vi "run_pharmaBotExp_v0.015.vi"(0 "data in":T12={"daq_ao 1"="Dev1/ao0", "daq_ai 1"="Dev1/ai0", "experiment day folder"=path "C:/multiBot/data/debug/testing", "Multiclamp init error"=0, "Multiclamp Handle Out"=10225184, "sampling rate (Hz)"=20000, "trial name"="t1"}, 1 "auto run?":bool=TRUE, 3 "which manipulator":T13(ring), 4 "HEK/slice options":enum16{"slice", "HEK"}(ring), 5 "error in":errorcluster, 6 "Validate after Experiment":bool, 7 "common cluster":T9, 11 "individual controls in":T8, 13 "images":T3={"slice image"="remote image 000000001461186C", "pipette template"="remote image 000000001461152C", "found pipette"=refnum, "pipette mask for cell tracker"=refnum, "cell images ref"=refnum}) -> (10 "Cell Looks Good?":bool=TRUE, 12 "ValidationOutputCluster":T5(array[cluster]), 14 "ValidationResults":waveform(dbl)[][](array[waveform]), 15 "ValidationPos1":T6(array[ring]), 16 "Exp. Terminated":bool, 17 "ValidationPos2":T6(array[ring]), 18 "ValidationWaveform":waveform(dbl)[](array[waveform]), 19 "error out":errorcluster)   [LabVIEW 2015] (continued)
          }
        }
        n1077 = Select(t="QualityCheck" ("ExpPhase"), s=w837, f="postLift" ("ExpPhase")) -> (s? t:f=w864:string)
        n1078 = call "run_repeatingMembraneTest_pharmabot.vi"("ExpPhase"=w864, "error in"=w900, "data in"=w899, "misc common.stop memtest"=w885, "controls array in"=w893) -> ("error out"=w897:errorcluster, "data out"=w898:T12, "Cell Good?"=w859:bool, "control array out"=w892:refnum<vi>[])  [unwired: 2 in, 1 out]
        n1079 = local write "Cell Looks Good?"(w859) -> ()
        n1080 = case shown="True" w859 {
          tunnel: w898 -> [w1208 w1260]
          tunnel: w897 -> [w1206 w1257]
          tunnel: w824 -> [_ w1235]
          tunnel: w833 -> [_ w1251]
          tunnel: w895 -> [_ w1250]
          tunnel: w894 -> [_ w1249]
          tunnel: w892 -> [w1203 w1248]
          tunnel: [w1208 w1244] -> w891
          tunnel: [w1205 w1225] -> w890
          tunnel: [w1204 w1226] -> w889
          tunnel: w885 -> [_ w1222]
          tunnel: w880 -> [_ w1241]
          tunnel: w879 -> [_ w1240]
          tunnel: w883 -> [w1201 _]
          tunnel: [w1195 w1231] -> w876
          tunnel: [w1198 w1233] -> w875
          tunnel: [w1194 w1232] -> w874
          tunnel: [w1196 w1230] -> w873
          tunnel: [w1197 w1229] -> w872
          tunnel: w837 -> [_ w1224]
          tunnel: w858 -> [_ w1218]
          frame False {
            n1081 = local read "ValidationOutputCluster"() -> (w1197:T5)
            n1082 = local read "ValidationWaveform"() -> (w1196:waveform(dbl)[])
            n1083 = local read "ValidationPos2"() -> (w1194:T6)
            n1084 = local read "ValidationPos1"() -> (w1198:T6)
            n1085 = local read "ValidationResults"() -> (w1195:waveform(dbl)[][])
            n1086 = call <vilib>:"Play Sound File.vi"("path"=path "C:/multiBot/patcherBot/sounds/Price_Is_Right_loser_clip.wav") -> ()  [unwired: 9 in, 2 out]
            n1087 = Select(t="Cell Lift Failed!" ("status string in"), s=w1201, f="Pulling Patch Failed!" ("status string in")) -> (s? t:f=w1202:string)
            n1088 = call "set_status_string.vi"("error in"=w1206, "new line?"=TRUE, "status string in"=w1202, "controls array"=w1203) -> ("error out"=w1205:errorcluster, "controls array out"=w1204:refnum<vi>[])  [unwired: 6 in]
          }
          frame True {
            n1089 = local read "How Many Experimental Phases?"() -> (w1234:i32)
            n1090 = local write "protocol creation"(T11."Experimental Procedures" ("protocol creation")) -> ()
            n1091 = case shown="True" w1224 {
              tunnel: w1257 -> [w1324 w1327]
              tunnel: [w1323 w1326] -> w1256
              tunnel: T42."Experiment Safe Position" ("Which Jumper Position to Set?") -> [w1322 _]
              tunnel: w1251 -> [w1321 _]
              tunnel: w1249 -> [w1320 _]
              tunnel: w1248 -> [w1319 w1329]
              tunnel: [w1318 w1328] -> w1247
              frame False {
                n1092 = call "moveToJumperPosition-v02.vi"("which manipulator"=w1320, "controls array in"=w1319, "Which Jumper Position to move to?"=w1322, "error in"=w1324, "common cluster"=w1321) -> ("control array out"=w1318:refnum<vi>[], "error out"=w1323:errorcluster)  [unwired: 9 in]
              }
              frame True {
                n1093 = call "set_status_string.vi"("error in"=w1327, "new line?"=TRUE, "status string in"="Not Moving", "controls array"=w1329) -> ("error out"=w1326:errorcluster, "controls array out"=w1328:refnum<vi>[])  [unwired: 6 in]
              }
            }
            n1094 = call "run_repeatingMembraneTest_pharmabot.vi"("ExpPhase"="preQC", "error in"=w1256, "data in"=w1260, "misc common.stop memtest"=w1222, "controls array in"=w1247) -> ("error out"=w1239:errorcluster, "data out"=w1258:T12, "Cell Good?"=w1221:bool, "control array out"=w1259:refnum<vi>[])  [unwired: 2 in, 1 out]
            n1095 = call "mclamp_zero_pipetteCap.vi"("error in (no error)"=w1239, "Error in"=w1240, "Multiclamp Handle Out"=w1241) -> ("error out"=w1238:errorcluster, "slow comp (pF)"=w1236:dbl, "fast comp (pF)"=w1237:dbl)  [unwired: 6 in]
            n1096 = local write "Cell Looks Good?"(w1221) -> ()
            n1097 = local write "slow comp (pF)"(w1236) -> ()
            n1098 = local write "fast comp (pF)"(w1237) -> ()
            n1099 = call "run_repeatingMembraneTest_pharmabot.vi"("ExpPhase"="preExp", "error in"=w1238, "data in"=w1258, "misc common.stop memtest"=w1222, "controls array in"=w1259) -> ("error out"=w1253:errorcluster, "data out"=w1245:T12, "Cell Good?"=w1220:bool, "control array out"=w1254:refnum<vi>[])  [unwired: 2 in, 1 out]
            n1100 = for {
              N: w1234 -> [_]
              tunnel: w1251 -> [w1334]
              tunnel: w1250 -> [w1335]
              tunnel: [w1345] -> w1246
              tunnel: w1254 -> [w1353]
              tunnel: w1249 -> [w1352]
              tunnel: w1235 -> [w1349]
              tunnel: w1253 -> [w1339]
              tunnel: [w1344] -> w1252
              tunnel: w1245 -> [w1350]
              tunnel: w1224 -> [w1348]
              shift-right: [w1346] -> _
              shift-left: FALSE ("Cell Good?") -> [w1347]
              tunnel: w1222 -> [w1343]
              tunnel: w1218 -> [w1342]
              tunnel: [w1332] -> w1217
              i -> [w1351]
              n1101 = Unbundle By Name(w1334) -> ("misc common.Terminate Experiment"=w1333:refnum<vi>)
              n1102 = control-ref of="Terminate Experiment"() -> (w1336:refnum<vi>)
              n1103 = control-ref of="Filtered currents (pA)"() -> (w1340:refnum<vi>)
              n1104 = property class="Bool (strict)"(reference=w1333) -> ("Value"=w1332:bool)  [unwired: 1 in, 2 out]
              n1105 = property class="WFGraph (strict)"(reference=w1340, error in=w1339, "Value"=waveform(dbl)[] []) -> (error out=w1338:errorcluster)  [unwired: 1 out]
              n1106 = property class="Bool (strict)"(reference=w1336, "Value"=w1332) -> ()  [unwired: 1 in, 2 out]
              n1107 = local read "current clamp"() -> (w1331:enum16{"VClamp", "IClamp"})
              n1108 = Or(x=w1332, y=w1347) -> (x .or. y?=w1341:bool)
              n1109 = case shown="False" w1341 {
                selector: w1341 -> [_ w1578]
                tunnel: w1334 -> [w1394 _]
                tunnel: w1335 -> [w1393 _]
                tunnel: w1353 -> [w1392 w1584]
                tunnel: w1352 -> [w1391 _]
                tunnel: w1338 -> [w1390 w1582]
                tunnel: w1351 -> [w1388 w1579]
                tunnel: w1350 -> [w1377 _]
                tunnel: w1349 -> [w1370 _]
                tunnel: w1348 -> [w1384 _]
                tunnel: [w1382 w1578] -> w1346
                tunnel: [w1379 w1577] -> w1345
                tunnel: [w1367 w1576] -> w1344
                tunnel: w1343 -> [w1376 _]
                tunnel: w1342 -> [w1371 _]
                tunnel: w1331 -> [w1358 _]
                frame False {
                  n1110 = Increment(x=w1388) -> (x+1=w1369:i32)
                  n1111 = case shown="1" w1369 {
                    tunnel: w1370 -> [w1502 w1508 w1514 w1520 w1526 w1532 w1538 w1544 w1550 w1556 w1562 w1568 w1574]
                    tunnel: [w1501 w1507 w1513 w1519 w1525 w1531 w1537 w1543 w1549 w1555 w1561 w1567 w1573] -> w1364
                    tunnel: w1390 -> [w1500 w1505 w1511 w1517 w1523 w1529 w1535 w1541 w1547 w1553 w1559 w1565 w1571]
                    tunnel: [w1500 w1505 w1511 w1517 w1523 w1529 w1535 w1541 w1547 w1553 w1559 w1565 w1571] -> w1389
                    tunnel: ["na" "A" "B" "C" "D" "E" "F" "G" "H" "I" "J" "K" "L"] -> w1355
                    tunnel: [w1498 w1504 w1510 w1516 w1522 w1528 w1534 w1540 w1546 w1552 w1558 w1564 w1570] -> w1361
                    tunnel: [T19."PhaseA" ("Experimental Phases") T19."PhaseA" ("Experimental Phases") T19."PhaseB" ("Experimental Phases") T19."PhaseC" ("Experimental Phases") T19."PhaseD" ("Experimental Phases") T19."PhaseE" ("Experimental Phases") T19."PhaseF" ("Experimental Phases") T19."PhaseG" ("Experimental Phases") T19."PhaseH" ("Experimental Phases") T19."PhaseI" ("Experimental Phases") T19."PhaseJ" ("Experimental Phases") T19."PhaseK" ("Experimental Phases") T19."PhaseL" ("Experimental Phases")] -> w1359
                    frame 0, Default {
                      n1112 = control-ref of="Experiment Selection A"() -> (w1498:refnum<vi>)
                      n1113 = Unbundle By Name(w1502) -> ("PhaseA Cluster"=w1501:T1)
                    }
                    frame 1 {
                      n1114 = Unbundle By Name(w1508) -> ("PhaseA Cluster"=w1507:T1)
                      n1115 = control-ref of="Experiment Selection A"() -> (w1504:refnum<vi>)
                    }
                    frame 2 {
                      n1116 = control-ref of="Experiment Selection B"() -> (w1510:refnum<vi>)
                      n1117 = Unbundle By Name(w1514) -> ("PhaseB Cluster"=w1513:T1)
                    }
                    frame 3 {
                      n1118 = Unbundle By Name(w1520) -> ("PhaseC Cluster"=w1519:T1)
                      n1119 = control-ref of="Experiment Selection C"() -> (w1516:refnum<vi>)
                    }
                    frame 4 {
                      n1120 = Unbundle By Name(w1526) -> ("PhaseD Cluster"=w1525:T1)
                      n1121 = control-ref of="Experiment Selection D"() -> (w1522:refnum<vi>)
                    }
                    frame 5 {
                      n1122 = Unbundle By Name(w1532) -> ("PhaseE Cluster"=w1531:T1)
                      n1123 = control-ref of="Experiment Selection E"() -> (w1528:refnum<vi>)
                    }
                    frame 6 {
                      n1124 = Unbundle By Name(w1538) -> ("PhaseF Cluster"=w1537:T1)
                      n1125 = control-ref of="Experiment Selection F"() -> (w1534:refnum<vi>)
                    }
                    frame 7 {
                      n1126 = control-ref of="Experiment Selection G"() -> (w1540:refnum<vi>)
                      n1127 = Unbundle By Name(w1544) -> ("PhaseG Cluster"=w1543:T1)
                    }
                    frame 8 {
                      n1128 = control-ref of="Experiment Selection H"() -> (w1546:refnum<vi>)
                      n1129 = Unbundle By Name(w1550) -> ("PhaseH Cluster"=w1549:T1)
                    }
                    frame 9 {
                      n1130 = control-ref of="Experiment Selection I"() -> (w1552:refnum<vi>)
                      n1131 = Unbundle By Name(w1556) -> ("PhaseI Cluster"=w1555:T1)
                    }
                    frame 10 {
                      n1132 = control-ref of="Experiment Selection J"() -> (w1558:refnum<vi>)
                      n1133 = Unbundle By Name(w1562) -> ("PhaseJ Cluster"=w1561:T1)
                    }
                    frame 11 {
                      n1134 = control-ref of="Experiment Selection K"() -> (w1564:refnum<vi>)
                      n1135 = Unbundle By Name(w1568) -> ("PhaseK Cluster"=w1567:T1)
                    }
                    frame 12 {
                      n1136 = Unbundle By Name(w1574) -> ("PhaseL Cluster"=w1573:T1)
                      n1137 = control-ref of="Experiment Selection L"() -> (w1570:refnum<vi>)
                    }
                  }
                  n1138 = Unbundle By Name(w1364) -> ("Phase Experiment Option"=w1363:refnum<vi>)
                  n1139 = property class="CmbBox"(reference=w1363) -> ("Value"=w1362:string)  [unwired: 1 in, 2 out]
                  n1140 = case shown="\"Current Pulse\"" w1362 {
                    tunnel: [T20."Single Jump" ("Value") T20."Solution Change" ("Value") T20."Voltage Step" ("Value") T20."Voltage Ramp" ("Value") T20."Voltage Pulse" ("Value") T20."Jump Train" ("Value") T20."Paired Pulse" ("Value") T20."Single Manip Jump" ("Value") T20."Gap Free" ("Value") T20."Multi M. Jump" ("Value") T20."Current Pulse" ("Value") T20."Current Ramp" ("Value") T20."Gap Free Iclamp" ("Value")] -> w1354
                    frame "Single Jump", Default {
                    }
                    frame "Solution Change" {
                    }
                    frame "Voltage Step" {
                    }
                    frame "Voltage Ramp" {
                    }
                    frame "Voltage Pulse" {
                    }
                    frame "Jump Train" {
                    }
                    frame "Paired Pulse" {
                    }
                    frame "Single Manip Jump" {
                    }
                    frame "Gap Free" {
                    }
                    frame "Multi M. Jump" {
                    }
                    frame "Current Pulse" {
                    }
                    frame "Current Ramp" {
                    }
                    frame "Gap Free Iclamp" {
                    }
                  }
                  n1141 = Unbundle By Name(w1370) -> ("time to wait for solution change (min)"=w1387:refnum<vi>, "valve Time Cluster"=w1385:T35)
                  n1142 = property class="DigNum (strict)"(reference=w1387) -> ("Value"=w1386:dbl)  [unwired: 1 in, 2 out]
                  n1143 = call "run_experiment_pharmaBot_v0.06.vi"("PhaseX Cluster"=w1364, "PhaseState"=w1355, "current clamp"=w1358, "time to wait for solution change (min)"=w1386, "valve Time Cluster"=w1385, "error in"=w1389, "which manipulator"=w1391, "common cluster"=w1394, "Didn't Lift?"=w1384, "controls array"=w1392, "individual controls in"=w1393, "data in"=w1377) -> ("control array out"=w1380:refnum<vi>[], "protocol response"=w1383:waveform(dbl)[], "set clamp"=w1357:enum16{"VClamp", "IClamp"}, "error out"=w1378:errorcluster)  [unwired: 3 in, 1 out]
                  n1144 = for {
                    tunnel: w1383 -> [w1448] mode=indexing
                    tunnel: [w1447] -> w1381 mode=indexing
                    tunnel: w1371 -> [w1449]
                    n1145 = in-place {
                      in-place-border: w1449 -> [w1460]
                      n1146 = in-place-cluster #1(w1448) -> ("Y"=w1455:dbl[])
                      n1147 = Index Array(array=w1455, index=0) -> (element=w1450:dbl)
                      n1148 = Subtract(x=w1455, y=w1450) -> (x-y=w1453:dbl[])
                      n1149 = call-poly <vilib>:"Bessel Filter.vi"("init/cont (init:F)"=TRUE, "order"=8, "filter type"=Filter_Passband_Type."Lowpass", "low cutoff freq: fl"=1000.0 ("sampling freq: fs"), "sampling freq: fs"=w1460, "X"=w1453) -> ("Filtered X"=w1451:dbl[])  [unwired: 2 in, 1 out]
                      n1150 = Add(x=w1451, y=w1450) -> (x+y=w1452:dbl[])
                      n1151 = in-place-cluster #1("Y"=w1452) -> (w1447:waveform(dbl))
                    }
                  }
                  n1152 = local write "current clamp"(w1357) -> ()
                  n1153 = local write "Filtered currents (pA)"(w1381) -> ()
                  n1154 = local write "Experimental Phases"(w1359) -> ()
                  n1155 = property class="TabCtl (strict)"(reference=w1361, "Value"=w1354) -> ()  [unwired: 1 in, 2 out]
                  n1156 = property class="TabCtl (strict)"(reference=w1361, "Visible"=TRUE) -> ()  [unwired: 1 in, 2 out]
                  n1157 = local read "Detect Recording Deterioration?"() -> (w1373:bool)
                  n1158 = Concatenate Strings("After Phase " ("string"), w1355) -> (w1374:string)
                  n1159 = call "run_repeatingMembraneTest_pharmabot.vi"("ExpPhase"=w1374, "error in"=w1378, "data in"=w1377, "misc common.stop memtest"=w1376, "controls array in"=w1380) -> ("error out"=w1368:errorcluster, "Cell Good?"=w1372:bool, "control array out"=w1379:refnum<vi>[], "cell stats"=w1356:T10)  [unwired: 2 in, 1 out]
                  n1160 = case shown="1" w1369 {
                    tunnel: w1370 -> [w1410 w1413 w1416 w1419 w1422 w1425 w1428 w1431 w1434 w1437 w1440 w1443 w1446]
                    tunnel: w1368 -> [w1409 w1412 w1415 w1418 w1421 w1424 w1427 w1430 w1433 w1436 w1439 w1442 w1445]
                    tunnel: [w1409 w1412 w1415 w1418 w1421 w1424 w1427 w1430 w1433 w1436 w1439 w1442 w1445] -> w1367
                    tunnel: [w1408 w1411 w1414 w1417 w1420 w1423 w1426 w1429 w1432 w1435 w1438 w1441 w1444] -> w1366
                    frame 0, Default {
                      n1161 = Unbundle By Name(w1410) -> ("PhaseStatusCluster.Phase L Done"=w1408:refnum<vi>)
                    }
                    frame 1 {
                      n1162 = Unbundle By Name(w1413) -> ("PhaseStatusCluster.Phase A Done"=w1411:refnum<vi>)
                    }
                    frame 2 {
                      n1163 = Unbundle By Name(w1416) -> ("PhaseStatusCluster.Phase B Done"=w1414:refnum<vi>)
                    }
                    frame 3 {
                      n1164 = Unbundle By Name(w1419) -> ("PhaseStatusCluster.Phase C Done"=w1417:refnum<vi>)
                    }
                    frame 4 {
                      n1165 = Unbundle By Name(w1422) -> ("PhaseStatusCluster.Phase D Done"=w1420:refnum<vi>)
                    }
                    frame 5 {
                      n1166 = Unbundle By Name(w1425) -> ("PhaseStatusCluster.Phase E Done"=w1423:refnum<vi>)
                    }
                    frame 6 {
                      n1167 = Unbundle By Name(w1428) -> ("PhaseStatusCluster.Phase F Done"=w1426:refnum<vi>)
                    }
                    frame 7 {
                      n1168 = Unbundle By Name(w1431) -> ("PhaseStatusCluster.Phase G Done"=w1429:refnum<vi>)
                    }
                    frame 8 {
                      n1169 = Unbundle By Name(w1434) -> ("PhaseStatusCluster.Phase H Done"=w1432:refnum<vi>)
                    }
                    frame 9 {
                      n1170 = Unbundle By Name(w1437) -> ("PhaseStatusCluster.Phase I Done"=w1435:refnum<vi>)
                    }
                    frame 10 {
                      n1171 = Unbundle By Name(w1440) -> ("PhaseStatusCluster.Phase J Done"=w1438:refnum<vi>)
                    }
                    frame 11 {
                      n1172 = Unbundle By Name(w1443) -> ("PhaseStatusCluster.Phase K Done"=w1441:refnum<vi>)
                    }
                    frame 12 {
                      n1173 = Unbundle By Name(w1446) -> ("PhaseStatusCluster.Phase L Done"=w1444:refnum<vi>)
                    }
                  }
                  n1174 = case shown="True" w1373 {
                    tunnel: [FALSE w1466] -> w1382
                    tunnel: w1372 -> [_ w1465]
                    tunnel: w1356 -> [_ w1464]
                    tunnel: w1355 -> [_ w1463]
                    tunnel: w1354 -> [_ w1462]
                    frame False {
                    }
                    frame True {
                      n1175 = case shown="False" w1465 {
                        tunnel: [w1471 FALSE ("T button?")] -> w1466
                        tunnel: w1464 -> [w1469 _]
                        tunnel: w1463 -> [w1468 _]
                        tunnel: w1462 -> [w1467 _]
                        frame False {
                          n1176 = local read "twitter?"() -> (w1470:bool)
                          n1177 = case shown="False" w1470 {
                            tunnel: [w1475 w1495] -> w1471
                            tunnel: w1469 -> [_ w1492]
                            tunnel: w1468 -> [_ w1494]
                            tunnel: w1467 -> [_ w1493]
                            frame False {
                              n1178 = Two Button Dialog(message="Cell Seal looks Questionable", 1:"Continue With Experiment" ("T button name (\"OK\")"), 2:"Terminate Experiment" ("T button name (\"OK\")")) -> (T button?=w1475:bool)
                              n1179 = call <vilib>:"Play Sound File.vi"("path"=path "C:/multiBot/patcherBot/sounds/wlk-yourmajesty.wav") -> ()  [unwired: 9 in, 2 out]
                              n1180 = call "jsontest.vi"("string"="Current Seal Looks Questionable send help!!!") -> ()  [unwired: 10 in, 1 out]
                            }
                            frame True {
                              n1181 = Current VI's Path() -> (path=w1480:path)
                              n1182 = Strip Path(path=w1480) -> (stripped path=w1490:path)  [unwired: 1 out]
                              n1183 = Strip Path(path=w1490) -> (stripped path=w1491:path)  [unwired: 1 out]
                              n1184 = Build Path(base path=w1491, name or relative path="test twitter command\\twitterSkipRemainingPhases.vi") -> (appended path=w1482:path)
                              n1185 = Open VI Reference(vi path=w1482) -> (vi reference=w1483:refnum<vi>, error out=w1484:errorcluster)  [unwired: 5 in]
                              n1186 = invoke class="VI" method="FP.Open"(reference=w1483, error in=w1484, "Activate"=TRUE ("Activate?"), "State"=T44."Standard") -> (reference out=w1489:refnum<vi>, error out=w1479:errorcluster)  [unwired: 1 in, 3 out]
                              n1187 = call "twitterSkipRemainingPhases.vi"("error in"=w1479, "Prev Exp"=w1493, "cell stats"=w1492, "Prev Phase"=w1494) -> ("error out"=w1478:errorcluster, "Skip Remaining"=w1495:bool)  [unwired: 6 in]
                              n1188 = invoke class="VI" method="FP.Close"(reference=w1489, error in=w1478) -> (reference out=w1487:refnum<vi>, error out=w1488:errorcluster)  [unwired: 1 in, 1 out]
                              n1189 = Close Reference(reference=w1487, error in (no error)=w1488) -> ()  [unwired: 1 out]
                            }
                          }
                        }
                        frame True {
                        }
                      }
                    }
                  }
                  n1190 = local write "Cell Looks Good?"(w1372) -> ()
                  n1191 = property class="Bool (strict)"(reference=w1366, "Value"=TRUE) -> ()  [unwired: 1 in, 2 out]
                }
                frame True {
                  n1192 = Increment(x=w1579) -> (x+1=w1575:i32)
                  n1193 = case shown="12" w1575 {
                    tunnel: w1582 -> [w1588 w1589 w1591 w1593 w1595 w1597 w1599 w1601 w1603 w1605 w1607 w1609 w1611]
                    tunnel: [w1588 w1589 w1591 w1593 w1595 w1597 w1599 w1601 w1603 w1605 w1607 w1609 w1611] -> w1583
                    tunnel: ["na" "A" "B" "C" "D" "E" "F" "G" "H" "I" "J" "K" "L"] -> w1580
                    frame 0, Default {
                    }
                    frame 1 {
                    }
                    frame 2 {
                    }
                    frame 3 {
                    }
                    frame 4 {
                    }
                    frame 5 {
                    }
                    frame 6 {
                    }
                    frame 7 {
                    }
                    frame 8 {
                    }
                    frame 9 {
                    }
                    frame 10 {
                    }
                    frame 11 {
                    }
                    frame 12 {
                    }
                  }
                  n1194 = Concatenate Strings("Skipped Phase" ("status string in"), w1580) -> (w1581:string)
                  n1195 = call "set_status_string.vi"("error in"=w1583, "new line?"=TRUE, "status string in"=w1581, "controls array"=w1584) -> ("error out"=w1576:errorcluster, "controls array out"=w1577:refnum<vi>[])  [unwired: 6 in]
                }
              }
            }
            n1196 = local write "Cell Looks Good?"(w1220) -> ()
            n1197 = call "Time Delay2"("error in (no error)"=w1252, "Delay Time (s)"=1.0) -> ("error out"=w1243:errorcluster)  [unwired: 9 in]
            n1198 = call "run_repeatingMembraneTest_pharmabot.vi"("ExpPhase"="postExp", "error in"=w1243, "data in"=w1245, "misc common.stop memtest"=w1222, "controls array in"=w1246) -> ("error out"=w1227:errorcluster, "data out"=w1244:T12, "Cell Good?"=w1219:bool, "control array out"=w1228:refnum<vi>[])  [unwired: 2 in, 1 out]
            n1199 = local write "Cell Looks Good?"(w1219) -> ()
            n1200 = local write "Exp. Terminated"(w1217) -> ()
            n1201 = local read "Validate after Experiment"() -> (w1210:bool)
            n1202 = control-ref of="Recorded currents (pA)"() -> (w1215:refnum<vi>)
            n1203 = control-ref of="Command steps (mV)"() -> (w1214:refnum<vi>)
            n1204 = Select(t=FALSE, s=w1224, f=w1210) -> (s? t:f=w1211:bool)
            n1205 = Bundle(cluster="Graph cluster", "Recorded currents (pA)"=w1215, "Command steps (mV)"=w1214) -> (w1212:T7)
            n1206 = case shown="True" w1211 {
              tunnel: w1251 -> [_ w1316]
              tunnel: w1250 -> [w1279 w1315]
              tunnel: w1249 -> [_ w1314]
              tunnel: w1244 -> [_ w1313]
              tunnel: w1212 -> [_ w1312]
              tunnel: w1228 -> [w1276 w1298]
              tunnel: w1227 -> [w1270 w1304]
              tunnel: [w1286 w1300] -> w1225
              tunnel: [w1285 w1295] -> w1226
              tunnel: w1235 -> [_ w1294]
              tunnel: [w1290 w1311] -> w1233
              tunnel: [w1289 w1310] -> w1232
              tunnel: [w1291 w1309] -> w1231
              tunnel: [w1292 w1308] -> w1230
              tunnel: [T5 [] ("ValidationOutputCluster") w1307] -> w1229
              frame False {
                w1282 = TRUE ("Set Status")
                w1284 = u16 1 ("ChangeToValve")
                # "valve 2"
                # "valve 1"
                n1207 = Unbundle By Name(w1279) -> ("misc indiv.daq_do 1"=w1278:tag, "misc indiv.daq_do 2"=w1277:tag, "misc indiv.V1-State"=w1272:refnum<vi>, "misc indiv.V2-State"=w1271:refnum<vi>)
                n1208 = property class="DigNum (strict)"(reference=w1272, error in=w1270) -> (error out=w1269:errorcluster, "Value"=w1274:u16)  [unwired: 1 out]
                n1209 = property class="DigNum (strict)"(reference=w1271, error in=w1269) -> (error out=w1268:errorcluster, "Value"=w1273:u16)  [unwired: 1 out]
                n1210 = call "sendValveSignal-v02.2.vi"("daq_do"=w1278, "Valve1?"=w1282, "ChangeToValve"=w1284, "CurrentValve"=w1274, "controls array in"=w1276, "Set Status"=w1282, "error in"=w1268) -> ("ValveSetTo"=w1280:u16, "error out"=w1267:errorcluster, "control array out"=w1283:refnum<vi>[])  [unwired: 5 in, 1 out]
                n1211 = call "sendValveSignal-v02.2.vi"("daq_do"=w1277, "ChangeToValve"=w1284, "CurrentValve"=w1273, "controls array in"=w1283, "Set Status"=w1282, "error in"=w1267) -> ("ValveSetTo"=w1281:u16, "error out"=w1266:errorcluster, "control array out"=w1275:refnum<vi>[])  [unwired: 6 in, 1 out]
                n1212 = property class="DigNum (strict)"(reference=w1272, error in=w1266, "Value"=w1280) -> (error out=w1265:errorcluster)  [unwired: 1 out]
                n1213 = property class="DigNum (strict)"(reference=w1271, error in=w1265, "Value"=w1281) -> (error out=w1264:errorcluster)  [unwired: 1 out]
                n1214 = call "set_status_string.vi"("error in"=w1264, "new line?"=TRUE, "status string in"="Skipped Validation", "controls array"=w1275) -> ("error out"=w1286:errorcluster, "controls array out"=w1285:refnum<vi>[])  [unwired: 6 in]
                n1215 = local read "ValidationWaveform"() -> (w1292:waveform(dbl)[])
                n1216 = local read "ValidationPos2"() -> (w1289:T6)
                n1217 = local read "ValidationPos1"() -> (w1290:T6)
                n1218 = local read "ValidationResults"() -> (w1291:waveform(dbl)[][])
              }
              frame True {
                # "blow out cell?"
                n1219 = call "set_status_string.vi"("error in"=w1304, "new line?"=TRUE, "status string in"="Starting Valudation", "controls array"=w1298) -> ("error out"=w1303:errorcluster, "controls array out"=w1297:refnum<vi>[])  [unwired: 6 in]
                n1220 = call "validate_experiment_pharmaBot_v0.06.vi"("ExperimentOptionsCluster"=w1294, "Open Tip?"=TRUE, "Graph cluster"=w1312, "error in"=w1303, "which manipulator"=w1314, "common cluster"=w1316, "controls array"=w1297, "individual controls in"=w1315, "data in"=w1313) -> ("control array out"=w1296:refnum<vi>[], "ValidationWaveform"=w1308:waveform(dbl)[], "ValidationResults"=w1309:waveform(dbl)[][], "ValidationPos1"=w1311:T6, "ValidationPos2"=w1310:T6, "ValidationOutputCluster"=w1307:T5, "error out"=w1299:errorcluster)  [unwired: 10 in, 2 out]
                n1221 = call "set_status_string.vi"("error in"=w1299, "new line?"=TRUE, "status string in"="Finished Validation", "controls array"=w1296) -> ("error out"=w1300:errorcluster, "controls array out"=w1295:refnum<vi>[])  [unwired: 6 in]
              }
            }
          }
        }
        "ValidationResults" <- w876
        "ValidationPos1" <- w875
        "ValidationPos2" <- w874
        "ValidationWaveform" <- w873
        "ValidationOutputCluster" <- w872
        n1222 = call "set_status_string.vi"("error in"=w890, "new line?"=TRUE, "status string in"="~~~AUTO RUN DONE~~~", "controls array"=w889) -> ("error out"=w834:errorcluster)  [unwired: 6 in, 1 out]
        n1223 = Unbundle By Name(w891) -> ("experiment day folder"=w887:path, "trial name"=w886:string)
        n1224 = Build Path(base path=w887, name or relative path=w886) -> (appended path=w884:path)
        n1225 = case shown="True" TRUE {
          tunnel: [TRUE ("Experiment Done") w924] -> w888
          tunnel: w884 -> [_ w923]
          tunnel: [w905 w911] -> w835
          tunnel: w834 -> [w905 w911]
          tunnel: w833 -> [_ w908]
          frame False {
          }
          frame True {
            w907 = FALSE ("Experiment Done")
            w924 = TRUE ("Experiment Done")
            n1226 = Unbundle By Name(w908) -> ("misc common.Terminate Experiment"=w909:refnum<vi>)
            n1227 = property class="Bool (strict)"(reference=w909, "Value"=FALSE) -> ()  [unwired: 1 in, 2 out]
            n1228 = Build Path(base path=w923, name or relative path="status.txt") -> (appended path=w921:path)
            n1229 = control-ref of="status"() -> (w913:refnum<vi>)
            n1230 = local write "auto WC run trigger"(w907) -> ()
            n1231 = local write "Exp Started"(w907) -> ()
            n1232 = local write "Experiment Done"(w924) -> ()
            n1233 = local write "Running"(w907) -> ()
            n1234 = property class="Str"(reference=w913) -> ("Value"=w912:string)  [unwired: 1 in, 2 out]
            n1235 = Open/Create/Replace File(file path (use dialog)=w921, operation (0:open)=T41."replace or create", access (0:read/write)=enum16{"read/write", "read-only", "write-only"}."read/write") -> (refnum out=w917:refnum<file>, error out=w918:errorcluster)  [unwired: 3 in, 1 out]
            n1236 = Write to Text File(file (use dialog)=w917, text=w912, error in=w918) -> (refnum out=w915:refnum<file>, error out=w916:errorcluster)  [unwired: 1 in, 1 out]
            n1237 = Wait (ms)(milliseconds to wait=u32 200) -> ()  [unwired: 1 out]
            n1238 = Close File(refnum=w915, error in=w916) -> ()  [unwired: 2 out]
          }
        }
      }
    }
    "error out" <- w796
    n1239 = Or(x=w804, y="stop") -> (x .or. y?=w805:bool)
    n1240 = Request Deallocation(TRUE ("flag")) -> ()
    n1241 = Wait (ms)(milliseconds to wait=u32 50) -> ()  [unwired: 1 out]
  }
  n1242 = while {
    tunnel: "protocol config" -> [w1616]
    tunnel: w474 -> [w1615]
    tunnel: w78 -> [w1613]
    stop <- w1614 stop-if-true
    n1243 = event shown="[5] \"Single Manip Jump A\", \"Single Manip Jump B\", \"Single Manip Jump C\", \"Single Manip Jump D\", \"Single Manip Jump E\", \"Single Manip Jump F\", \"Single Manip Jump L\", \"Single Manip Jump K\", \"Single Manip Jump J\", \"Single Manip Jump I\", \"Single Manip Jump H\", \"Single Manip Jump G\": Value Change" {
      selector: _ -> [_ _ _ _ _ _ _ _ _ _ _ _ _ _ _ _ _ _ _ _ _ _]
      dyn-events: _ -> [_ _ _ _ _ _ _ _ _ _ _ _ _ _ _ _ _ _ _ _ _ _]
      timeout: _ -> [_ _ _ _ _ _ _ _ _ _ _ _ _ _ _ _ _ _ _ _ _ _]
      tunnel: w1616 -> [_ _ _ _ _ _ _ _ _ _ _ _ _ _ _ _ _ _ _ _ w3159 _]
      tunnel: w1615 -> [_ _ _ _ _ _ _ _ _ _ _ _ _ _ _ _ _ _ _ _ w3158 w3209]
      tunnel: [w1617 w1695 _ FALSE ("NewVal") FALSE ("NewVal") _ _ _ _ _ _ _ _ _ _ _ w3051 TRUE ("NewVal") _ _ FALSE ("NewVal") FALSE ("NewVal")] -> w1614
      tunnel: w1613 -> [_ _ _ _ _ _ _ _ _ _ _ _ _ _ _ _ w3050 _ w3109 w3131 w3154 w3206]
      event Timeout {
        n1244 = event-data() -> ()  [unwired: 1 in, 3 out]
        n1245 = local read "Running"() -> (w1618:bool)
        n1246 = case shown="False" w1618 {
          tunnel: [w1620 FALSE] -> w1617
          frame False {
            n1247 = local read "Experiment Done"() -> (w1620:bool)
          }
          frame True {
          }
        }
        n1248 = Wait (ms)(milliseconds to wait=u32 50) -> ()  [unwired: 1 out]
      }
      event "stop": Value Change {
        n1249 = event-data() -> ("NewVal"=w1695:bool)  [unwired: 1 in, 5 out]
        n1250 = control-ref of="Experiment Selection B"() -> (w1690:refnum<vi>)
        n1251 = control-ref of="Experiment Selection C"() -> (w1689:refnum<vi>)
        n1252 = control-ref of="Experiment Selection D"() -> (w1684:refnum<vi>)
        n1253 = control-ref of="Experiment Selection A"() -> (w1693:refnum<vi>)
        n1254 = control-ref of="Experiment Selection F"() -> (w1682:refnum<vi>)
        n1255 = control-ref of="Experiment Selection E"() -> (w1683:refnum<vi>)
        n1256 = Wait (ms)(milliseconds to wait=u32 100) -> ()  [unwired: 1 out]
        n1257 = property class="TabCtl (strict)"(reference=w1684, "Tabs Visible?"=TRUE) -> ()  [unwired: 1 in, 2 out]
        n1258 = property class="TabCtl (strict)"(reference=w1683, "Tabs Visible?"=TRUE) -> ()  [unwired: 1 in, 2 out]
        n1259 = property class="TabCtl (strict)"(reference=w1682, "Tabs Visible?"=TRUE) -> ()  [unwired: 1 in, 2 out]
        n1260 = property class="TabCtl (strict)"(reference=w1689, "Tabs Visible?"=TRUE) -> ()  [unwired: 1 in, 2 out]
        n1261 = property class="TabCtl (strict)"(reference=w1690, "Tabs Visible?"=TRUE) -> ()  [unwired: 1 in, 2 out]
        n1262 = property class="TabCtl (strict)"(reference=w1693, "Tabs Visible?"=TRUE) -> ()  [unwired: 1 in, 2 out]
        n1263 = Not(x=w1695) -> (.not. x?=w1694:bool)
        n1264 = property on="Experiment Done" class="Bool (strict)"("Value"=w1695) -> ()  [unwired: 2 in, 2 out]
        n1265 = property on="Running" class="Bool (strict)"("Value"=w1694) -> ()  [unwired: 2 in, 2 out]
        n1266 = control-ref of="Experiment Selection L"() -> (w1681:refnum<vi>)
        n1267 = control-ref of="Experiment Selection K"() -> (w1680:refnum<vi>)
        n1268 = control-ref of="Experiment Selection H"() -> (w1673:refnum<vi>)
        n1269 = control-ref of="Experiment Selection I"() -> (w1674:refnum<vi>)
        n1270 = control-ref of="Experiment Selection G"() -> (w1670:refnum<vi>)
        n1271 = control-ref of="Experiment Selection J"() -> (w1679:refnum<vi>)
        n1272 = control-ref of="PhaseB Experiment Option"() -> (w1667:refnum<vi>)
        n1273 = control-ref of="PhaseF Experiment Option"() -> (w1649:refnum<vi>)
        n1274 = control-ref of="PhaseA Experiment Option"() -> (w1669:refnum<vi>)
        n1275 = control-ref of="PhaseD Experiment Option"() -> (w1657:refnum<vi>)
        n1276 = control-ref of="PhaseC Experiment Option"() -> (w1658:refnum<vi>)
        n1277 = control-ref of="PhaseE Experiment Option"() -> (w1650:refnum<vi>)
        n1278 = property class="TabCtl (strict)"(reference=w1681, "Tabs Visible?"=TRUE) -> ()  [unwired: 1 in, 2 out]
        n1279 = property class="TabCtl (strict)"(reference=w1680, "Tabs Visible?"=TRUE) -> ()  [unwired: 1 in, 2 out]
        n1280 = property class="TabCtl (strict)"(reference=w1679, "Tabs Visible?"=TRUE) -> ()  [unwired: 1 in, 2 out]
        n1281 = property class="TabCtl (strict)"(reference=w1674, "Tabs Visible?"=TRUE) -> ()  [unwired: 1 in, 2 out]
        n1282 = property class="TabCtl (strict)"(reference=w1673, "Tabs Visible?"=TRUE) -> ()  [unwired: 1 in, 2 out]
        n1283 = property class="TabCtl (strict)"(reference=w1670, "Tabs Visible?"=TRUE) -> ()  [unwired: 1 in, 2 out]
        n1284 = property class="CmbBox"(reference=w1669, "Visible"=TRUE) -> ()  [unwired: 1 in, 2 out]
        n1285 = property class="CmbBox"(reference=w1667, "Visible"=TRUE) -> ()  [unwired: 1 in, 2 out]
        n1286 = property class="CmbBox"(reference=w1649, "Visible"=TRUE) -> ()  [unwired: 1 in, 2 out]
        n1287 = property class="CmbBox"(reference=w1657, "Visible"=TRUE) -> ()  [unwired: 1 in, 2 out]
        n1288 = property class="CmbBox"(reference=w1658, "Visible"=TRUE) -> ()  [unwired: 1 in, 2 out]
        n1289 = property class="CmbBox"(reference=w1650, "Visible"=TRUE) -> ()  [unwired: 1 in, 2 out]
        n1290 = control-ref of="Experiment Selection B"() -> (w1664:refnum<vi>)
        n1291 = control-ref of="Experiment Selection F"() -> (w1646:refnum<vi>)
        n1292 = control-ref of="Experiment Selection D"() -> (w1654:refnum<vi>)
        n1293 = control-ref of="Experiment Selection A"() -> (w1662:refnum<vi>)
        n1294 = control-ref of="Experiment Selection C"() -> (w1661:refnum<vi>)
        n1295 = control-ref of="Experiment Selection E"() -> (w1653:refnum<vi>)
        n1296 = property class="TabCtl (strict)"(reference=w1664, "Visible"=TRUE) -> ()  [unwired: 1 in, 2 out]
        n1297 = property class="TabCtl (strict)"(reference=w1662, "Visible"=TRUE) -> ()  [unwired: 1 in, 2 out]
        n1298 = property class="TabCtl (strict)"(reference=w1646, "Visible"=TRUE) -> ()  [unwired: 1 in, 2 out]
        n1299 = property class="TabCtl (strict)"(reference=w1654, "Visible"=TRUE) -> ()  [unwired: 1 in, 2 out]
        n1300 = property class="TabCtl (strict)"(reference=w1661, "Visible"=TRUE) -> ()  [unwired: 1 in, 2 out]
        n1301 = property class="TabCtl (strict)"(reference=w1653, "Visible"=TRUE) -> ()  [unwired: 1 in, 2 out]
        n1302 = control-ref of="PhaseH Experiment Option"() -> (w1624:refnum<vi>)
        n1303 = control-ref of="PhaseL Experiment Option"() -> (w1642:refnum<vi>)
        n1304 = control-ref of="PhaseG Experiment Option"() -> (w1622:refnum<vi>)
        n1305 = control-ref of="PhaseJ Experiment Option"() -> (w1634:refnum<vi>)
        n1306 = control-ref of="PhaseI Experiment Option"() -> (w1633:refnum<vi>)
        n1307 = control-ref of="PhaseK Experiment Option"() -> (w1641:refnum<vi>)
        n1308 = property class="CmbBox"(reference=w1622, "Visible"=TRUE) -> ()  [unwired: 1 in, 2 out]
        n1309 = property class="CmbBox"(reference=w1624, "Visible"=TRUE) -> ()  [unwired: 1 in, 2 out]
        n1310 = property class="CmbBox"(reference=w1642, "Visible"=TRUE) -> ()  [unwired: 1 in, 2 out]
        n1311 = property class="CmbBox"(reference=w1634, "Visible"=TRUE) -> ()  [unwired: 1 in, 2 out]
        n1312 = property class="CmbBox"(reference=w1633, "Visible"=TRUE) -> ()  [unwired: 1 in, 2 out]
        n1313 = property class="CmbBox"(reference=w1641, "Visible"=TRUE) -> ()  [unwired: 1 in, 2 out]
        n1314 = control-ref of="Experiment Selection H"() -> (w1627:refnum<vi>)
        n1315 = control-ref of="Experiment Selection L"() -> (w1645:refnum<vi>)
        n1316 = control-ref of="Experiment Selection J"() -> (w1637:refnum<vi>)
        n1317 = control-ref of="Experiment Selection G"() -> (w1629:refnum<vi>)
        n1318 = control-ref of="Experiment Selection I"() -> (w1630:refnum<vi>)
        n1319 = control-ref of="Experiment Selection K"() -> (w1638:refnum<vi>)
        n1320 = property class="TabCtl (strict)"(reference=w1627, "Visible"=TRUE) -> ()  [unwired: 1 in, 2 out]
        n1321 = property class="TabCtl (strict)"(reference=w1629, "Visible"=TRUE) -> ()  [unwired: 1 in, 2 out]
        n1322 = property class="TabCtl (strict)"(reference=w1645, "Visible"=TRUE) -> ()  [unwired: 1 in, 2 out]
        n1323 = property class="TabCtl (strict)"(reference=w1637, "Visible"=TRUE) -> ()  [unwired: 1 in, 2 out]
        n1324 = property class="TabCtl (strict)"(reference=w1630, "Visible"=TRUE) -> ()  [unwired: 1 in, 2 out]
        n1325 = property class="TabCtl (strict)"(reference=w1638, "Visible"=TRUE) -> ()  [unwired: 1 in, 2 out]
      }
      event "Experiment Done": Value Change {
        n1326 = event-data() -> ()  [unwired: 1 in, 6 out]
        n1327 = control-ref of="Experiment Selection A"() -> (w1721:refnum<vi>)
        n1328 = control-ref of="Experiment Selection B"() -> (w1718:refnum<vi>)
        n1329 = control-ref of="Experiment Selection C"() -> (w1717:refnum<vi>)
        n1330 = control-ref of="Experiment Selection D"() -> (w1712:refnum<vi>)
        n1331 = control-ref of="Experiment Selection E"() -> (w1711:refnum<vi>)
        n1332 = control-ref of="Experiment Selection F"() -> (w1710:refnum<vi>)
        n1333 = property class="TabCtl (strict)"(reference=w1711, "Tabs Visible?"=TRUE) -> ()  [unwired: 1 in, 2 out]
        n1334 = property class="TabCtl (strict)"(reference=w1710, "Tabs Visible?"=TRUE) -> ()  [unwired: 1 in, 2 out]
        n1335 = property class="TabCtl (strict)"(reference=w1712, "Tabs Visible?"=TRUE) -> ()  [unwired: 1 in, 2 out]
        n1336 = property class="TabCtl (strict)"(reference=w1717, "Tabs Visible?"=TRUE) -> ()  [unwired: 1 in, 2 out]
        n1337 = property class="TabCtl (strict)"(reference=w1721, "Tabs Visible?"=TRUE) -> ()  [unwired: 1 in, 2 out]
        n1338 = property class="TabCtl (strict)"(reference=w1718, "Tabs Visible?"=TRUE) -> ()  [unwired: 1 in, 2 out]
        n1339 = control-ref of="Experiment Selection G"() -> (w1697:refnum<vi>)
        n1340 = control-ref of="Experiment Selection H"() -> (w1700:refnum<vi>)
        n1341 = control-ref of="Experiment Selection I"() -> (w1701:refnum<vi>)
        n1342 = control-ref of="Experiment Selection J"() -> (w1706:refnum<vi>)
        n1343 = control-ref of="Experiment Selection K"() -> (w1707:refnum<vi>)
        n1344 = control-ref of="Experiment Selection L"() -> (w1708:refnum<vi>)
        n1345 = Wait (ms)(milliseconds to wait=u32 100) -> ()  [unwired: 1 out]
        n1346 = property class="TabCtl (strict)"(reference=w1707, "Tabs Visible?"=TRUE) -> ()  [unwired: 1 in, 2 out]
        n1347 = property class="TabCtl (strict)"(reference=w1708, "Tabs Visible?"=TRUE) -> ()  [unwired: 1 in, 2 out]
        n1348 = property class="TabCtl (strict)"(reference=w1706, "Tabs Visible?"=TRUE) -> ()  [unwired: 1 in, 2 out]
        n1349 = property class="TabCtl (strict)"(reference=w1701, "Tabs Visible?"=TRUE) -> ()  [unwired: 1 in, 2 out]
        n1350 = property class="TabCtl (strict)"(reference=w1697, "Tabs Visible?"=TRUE) -> ()  [unwired: 1 in, 2 out]
        n1351 = property class="TabCtl (strict)"(reference=w1700, "Tabs Visible?"=TRUE) -> ()  [unwired: 1 in, 2 out]
      }
      event "PhaseA Experiment Option", "PhaseB Experiment Option", "PhaseC Experiment Option", "PhaseD Experiment Option", "PhaseE Experiment Option", "PhaseF Experiment Option", "PhaseG Experiment Option", "PhaseH Experiment Option", "PhaseI Experiment Option", "PhaseJ Experiment Option", "PhaseK Experiment Option", "PhaseL Experiment Option": Value Change {
        n1352 = event-data() -> ("CtlRef"=w1736:refnum<vi>, "NewVal"=w1735:string)  [unwired: 1 in, 4 out]
        n1353 = property class="CmbBox"(reference=w1736) -> ("Label.Text"=w1738:string)  [unwired: 1 in, 2 out]
        n1354 = case shown="\"PhaseL Experiment Option\"" w1738 {
          tunnel: w1735 -> [_ w1753 w1809 w1865 w1921 w1977 w2033 w2089 w2145 w2201 w2257 w2313 w2369]
          tunnel: T20."Multi M. Jump" ("Value") -> [_ w1751 w1807 w1863 w1919 w1975 w2031 w2087 w2143 w2199 w2255 w2311 w2367]
          tunnel: T20."Single Jump" ("Value") -> [_ w1750 w1806 w1862 w1918 w1974 w2030 w2086 w2142 w2198 w2254 w2310 w2366]
          tunnel: T20."Solution Change" ("Value") -> [_ w1749 w1805 w1861 w1917 w1973 w2029 w2085 w2141 w2197 w2253 w2309 w2365]
          tunnel: T20."Voltage Step" ("Value") -> [_ w1748 w1804 w1860 w1916 w1972 w2028 w2084 w2140 w2196 w2252 w2308 w2364]
          tunnel: T20."Voltage Ramp" ("Value") -> [_ w1747 w1803 w1859 w1915 w1971 w2027 w2083 w2139 w2195 w2251 w2307 w2363]
          tunnel: T20."Voltage Pulse" ("Value") -> [_ w1746 w1802 w1858 w1914 w1970 w2026 w2082 w2138 w2194 w2250 w2306 w2362]
          tunnel: T20."Jump Train" ("Value") -> [_ w1745 w1801 w1857 w1913 w1969 w2025 w2081 w2137 w2193 w2249 w2305 w2361]
          tunnel: T20."Paired Pulse" ("Value") -> [_ w1744 w1800 w1856 w1912 w1968 w2024 w2080 w2136 w2192 w2248 w2304 w2360]
          tunnel: T20."Single Manip Jump" ("Value") -> [_ w1743 w1799 w1855 w1911 w1967 w2023 w2079 w2135 w2191 w2247 w2303 w2359]
          tunnel: T20."Gap Free" ("Value") -> [_ w1742 w1798 w1854 w1910 w1966 w2022 w2078 w2134 w2190 w2246 w2302 w2358]
          tunnel: T20."Gap Free Iclamp" ("Value") -> [_ w1741 w1797 w1853 w1909 w1965 w2021 w2077 w2133 w2189 w2245 w2301 w2357]
          tunnel: T20."Current Pulse" ("Value") -> [_ w1740 w1796 w1852 w1908 w1964 w2020 w2076 w2132 w2188 w2244 w2300 w2356]
          tunnel: T20."Current Ramp" ("Value") -> [_ w1739 w1795 w1851 w1907 w1963 w2019 w2075 w2131 w2187 w2243 w2299 w2355]
          frame "Null", Default {
          }
          frame "PhaseA Experiment Option" {
            n1355 = control-ref of="Experiment Selection A"() -> (w1752:refnum<vi>)
            n1356 = case shown="\"Current Ramp\"" w1753 {
              tunnel: w1752 -> [_ w1755 w1758 w1761 w1764 w1767 w1770 w1773 w1776 w1779 w1782 w1785 w1788 w1791 w1793]
              tunnel: w1751 -> [_ _ _ _ _ _ _ _ _ _ _ _ _ w1790 _]
              tunnel: w1750 -> [_ w1754 _ _ _ _ _ _ _ _ _ _ _ _ _]
              tunnel: w1749 -> [_ _ w1757 _ _ _ _ _ _ _ _ _ _ _ _]
              tunnel: w1748 -> [_ _ _ w1760 _ _ _ _ _ _ _ _ _ _ _]
              tunnel: w1747 -> [_ _ _ _ w1763 _ _ _ _ _ _ _ _ _ _]
              tunnel: w1746 -> [_ _ _ _ _ w1766 _ _ _ _ _ _ _ _ _]
              tunnel: w1745 -> [_ _ _ _ _ _ w1769 _ _ _ _ _ _ _ _]
              tunnel: w1744 -> [_ _ _ _ _ _ _ w1772 _ _ _ _ _ _ _]
              tunnel: w1743 -> [_ _ _ _ _ _ _ _ w1775 _ _ _ _ _ _]
              tunnel: w1742 -> [_ _ _ _ _ _ _ _ _ w1778 _ _ _ _ _]
              tunnel: w1741 -> [_ _ _ _ _ _ _ _ _ _ w1781 _ _ _ _]
              tunnel: w1740 -> [_ _ _ _ _ _ _ _ _ _ _ w1784 _ _ _]
              tunnel: w1739 -> [_ _ _ _ _ _ _ _ _ _ _ _ w1787 _ _]
              frame "False", Default {
              }
              frame "Single Jump" {
                n1357 = property class="TabCtl (strict)"(reference=w1755, "Value"=w1754) -> ()  [unwired: 1 in, 2 out]
                n1358 = property class="TabCtl (strict)"(reference=w1755, "Visible"=TRUE) -> ()  [unwired: 1 in, 2 out]
              }
              frame "Solution Change" {
                n1359 = property class="TabCtl (strict)"(reference=w1758, "Visible"=TRUE) -> ()  [unwired: 1 in, 2 out]
                n1360 = property class="TabCtl (strict)"(reference=w1758, "Value"=w1757) -> ()  [unwired: 1 in, 2 out]
              }
              frame "Voltage Step" {
                n1361 = property class="TabCtl (strict)"(reference=w1761, "Value"=w1760) -> ()  [unwired: 1 in, 2 out]
                n1362 = property class="TabCtl (strict)"(reference=w1761, "Visible"=TRUE) -> ()  [unwired: 1 in, 2 out]
              }
              frame "Voltage Ramp" {
                n1363 = property class="TabCtl (strict)"(reference=w1764, "Value"=w1763) -> ()  [unwired: 1 in, 2 out]
                n1364 = property class="TabCtl (strict)"(reference=w1764, "Visible"=TRUE) -> ()  [unwired: 1 in, 2 out]
              }
              frame "Voltage Pulse" {
                n1365 = property class="TabCtl (strict)"(reference=w1767, "Value"=w1766) -> ()  [unwired: 1 in, 2 out]
                n1366 = property class="TabCtl (strict)"(reference=w1767, "Visible"=TRUE) -> ()  [unwired: 1 in, 2 out]
              }
              frame "Jump Train" {
                n1367 = property class="TabCtl (strict)"(reference=w1770, "Value"=w1769) -> ()  [unwired: 1 in, 2 out]
                n1368 = property class="TabCtl (strict)"(reference=w1770, "Visible"=TRUE) -> ()  [unwired: 1 in, 2 out]
              }
              frame "Paired Pulse" {
                n1369 = property class="TabCtl (strict)"(reference=w1773, "Value"=w1772) -> ()  [unwired: 1 in, 2 out]
                n1370 = property class="TabCtl (strict)"(reference=w1773, "Visible"=TRUE) -> ()  [unwired: 1 in, 2 out]
              }
              frame "Single Manip Jump" {
                n1371 = property class="TabCtl (strict)"(reference=w1776, "Value"=w1775) -> ()  [unwired: 1 in, 2 out]
                n1372 = property class="TabCtl (strict)"(reference=w1776, "Visible"=TRUE) -> ()  [unwired: 1 in, 2 out]
              }
              frame "Gap Free" {
                n1373 = property class="TabCtl (strict)"(reference=w1779, "Value"=w1778) -> ()  [unwired: 1 in, 2 out]
                n1374 = property class="TabCtl (strict)"(reference=w1779, "Visible"=TRUE) -> ()  [unwired: 1 in, 2 out]
              }
              frame "Gap Free Iclamp" {
                n1375 = property class="TabCtl (strict)"(reference=w1782, "Value"=w1781) -> ()  [unwired: 1 in, 2 out]
                n1376 = property class="TabCtl (strict)"(reference=w1782, "Visible"=TRUE) -> ()  [unwired: 1 in, 2 out]
              }
              frame "Current Pulse" {
                n1377 = property class="TabCtl (strict)"(reference=w1785, "Value"=w1784) -> ()  [unwired: 1 in, 2 out]
                n1378 = property class="TabCtl (strict)"(reference=w1785, "Visible"=TRUE) -> ()  [unwired: 1 in, 2 out]
              }
              frame "Current Ramp" {
                n1379 = property class="TabCtl (strict)"(reference=w1788, "Value"=w1787) -> ()  [unwired: 1 in, 2 out]
                n1380 = property class="TabCtl (strict)"(reference=w1788, "Visible"=TRUE) -> ()  [unwired: 1 in, 2 out]
              }
              frame "Multi M. Jump" {
                n1381 = property class="TabCtl (strict)"(reference=w1791, "Value"=w1790) -> ()  [unwired: 1 in, 2 out]
                n1382 = property class="TabCtl (strict)"(reference=w1791, "Visible"=TRUE) -> ()  [unwired: 1 in, 2 out]
              }
              frame "none" {
                n1383 = property class="TabCtl (strict)"(reference=w1793, "Visible"=FALSE) -> ()  [unwired: 1 in, 2 out]
              }
            }
          }
          frame "PhaseB Experiment Option" {
            n1384 = control-ref of="Experiment Selection B"() -> (w1808:refnum<vi>)
            n1385 = case shown="\"Current Ramp\"" w1809 {
              tunnel: w1808 -> [_ w1811 w1814 w1817 w1820 w1823 w1826 w1829 w1832 w1835 w1838 w1841 w1844 w1847 w1849]
              tunnel: w1807 -> [_ _ _ _ _ _ _ _ _ _ _ _ _ w1846 _]
              tunnel: w1806 -> [_ w1810 _ _ _ _ _ _ _ _ _ _ _ _ _]
              tunnel: w1805 -> [_ _ w1813 _ _ _ _ _ _ _ _ _ _ _ _]
              tunnel: w1804 -> [_ _ _ w1816 _ _ _ _ _ _ _ _ _ _ _]
              tunnel: w1803 -> [_ _ _ _ w1819 _ _ _ _ _ _ _ _ _ _]
              tunnel: w1802 -> [_ _ _ _ _ w1822 _ _ _ _ _ _ _ _ _]
              tunnel: w1801 -> [_ _ _ _ _ _ w1825 _ _ _ _ _ _ _ _]
              tunnel: w1800 -> [_ _ _ _ _ _ _ w1828 _ _ _ _ _ _ _]
              tunnel: w1799 -> [_ _ _ _ _ _ _ _ w1831 _ _ _ _ _ _]